vi "Step-3-Top.vi"(9 "Override Iterations":bool=TRUE, 10 "# of Iterations":i32, 11 "input":T1={"a"=[17305248937841088298, 17024460552111218704], "b"=[9581029972675991065, 9654787791092207119], "hp_state_in"=array[2097152 elements], "hp_state_out"=array[2097152 elements], "hp_state_in (u64)"=array[262144 elements], "hp_state_out (u64)"=array[262144 elements]} {"a" format="%.0x"; "b" format="%.0x"; "hp_state_in" format="%.0x"; "hp_state_out" format="%.0x"; "hp_state_in (u64)" format="%.0x"; "hp_state_out (u64)" format="%.0x"}) -> (0 "hp_state out (u64)":u64[](array[numeric]) format="%.0x", 2 "b_out":u64[](array[numeric]) format="%.0x", 3 "a_out":u64[](array[numeric]) format="%.0x")   [LabVIEW 2017]
uses:
  Tests/Helpers/Step-3-Data-Type.ctl
panel:
  out "# of Iterations":i32
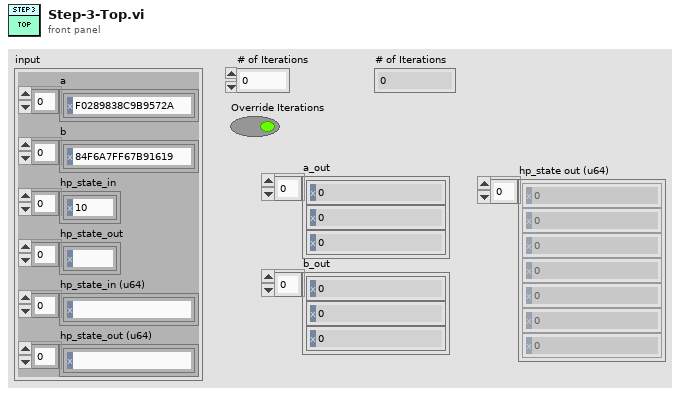
[diagram p1: front panel]
types:
  T1 = typedef "Step-3-Data-Type.ctl" = cluster{"a":u64[], "b":u64[], "hp_state_in":u8[], "hp_state_out":u8[], "hp_state_in (u64)":u64[], "hp_state_out (u64)":u64[]}
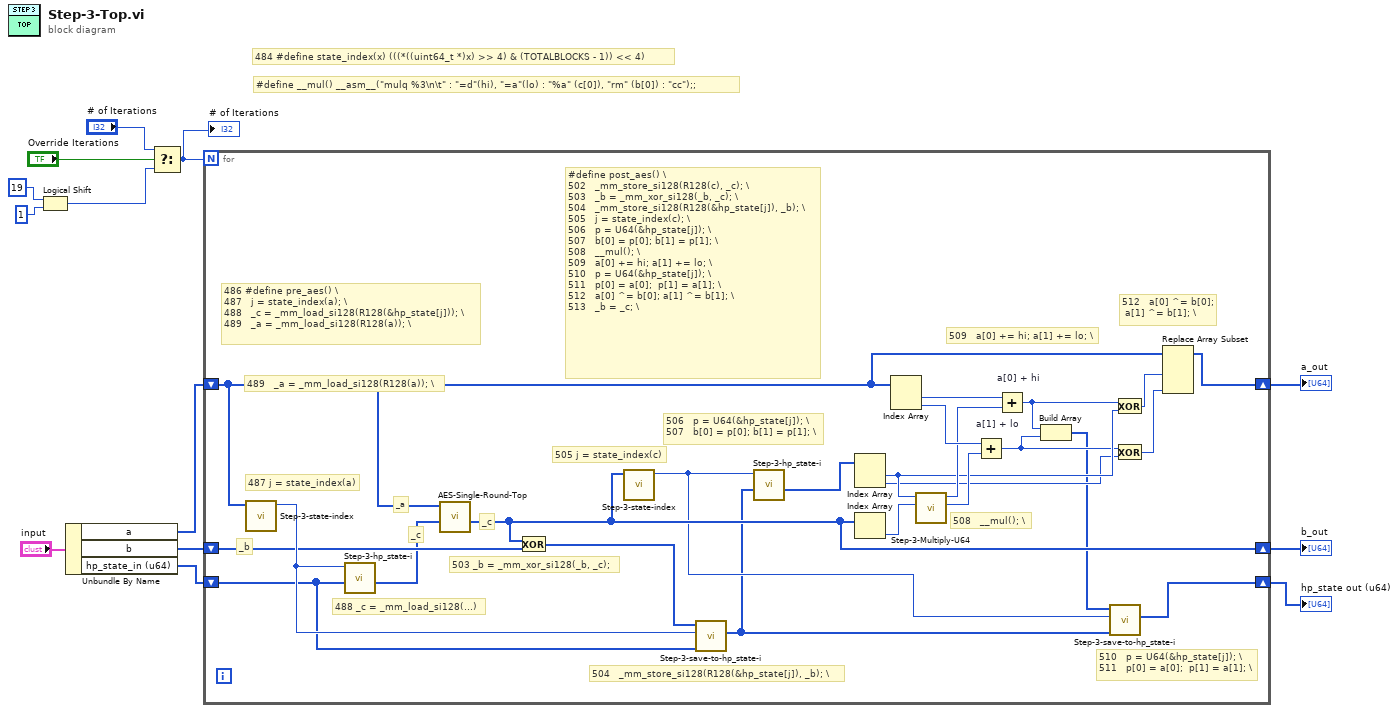
[diagram p0: block diagram]
diagram:
  # "#define __mul() __asm__(\"mulq %3\\n\\t\" : \"=d\"(hi), \"=a\"(lo) : \"%a\" (c[0]), \"rm\" (b[0]) : \"cc\");;"
  # "484 #define state_index(x) (((*((uint64_t *)x) >> 4) & (TOTALBLOCKS - 1)) << 4)"
  n1 = Logical Shift(y=19, x=1) -> (x << y=w6:i32)
  n2 = Unbundle By Name("input") -> ("a"=w11:u64[], "b"=w10:u64[], "hp_state_in (u64)"=w2:u64[])
  n3 = Select(t="# of Iterations", s="Override Iterations", f=w6) -> (s? t:f=w4:i32)
  "# of Iterations" <- w4
  n4 = for {
    N: w4 -> [_]
    shift-right: [w26] -> w9
    shift-left: w10 -> [w29]
    shift-right: [w31] -> w8
    shift-left: w11 -> [w14]
    shift-right: [w17] -> w1
    shift-left: w2 -> [w23]
    # "_c"
    # "_a"
    # "489   _a = _mm_load_si128(R128(a)); \\"
    # "510   p = U64(&hp_state[j]); \\\n511   p[0] = a[0];  p[1] = a[1]; \\"
    # "508   __mul(); \\"
    # "509   a[0] += hi; a[1] += lo; \\"
    # "512   a[0] ^= b[0];\n a[1] ^= b[1]; \\"
    # "506   p = U64(&hp_state[j]); \\\n507   b[0] = p[0]; b[1] = p[1]; \\"
    # "505 j = state_index(c)"
    # "504   _mm_store_si128(R128(&hp_state[j]), _b); \\"
    # "_c"
    # "_b"
    # "503 _b = _mm_xor_si128(_b, _c);"
    # "488 _c = _mm_load_si128(...)"
    # "487 j = state_index(a)"
    # "#define post_aes() \\\n502   _mm_store_si128(R128(c), _c); \\\n503   _b = _mm_xor_si128(_b, _c); \\\n504   _mm_store_si128(R128(&hp_state[j]), _b); \\\n505   j = state_index(c); \\\n506   p = U64(&hp_state[j]); \\\n507   b[0] = p[0]; b[1] = p[1]; \\\n508   __mul(); \\\n509   a[0] += hi; a[1] += lo; \\\n510   p = U64(&hp_state[j]); \\\n511   p[0] = a[0];  p[1] = a[1]; \\\n512   a[0] ^= b[0]; a[1] ^= b[1]; \\\n513   _b = _c; \\"
    # "486 #define pre_aes() \\\n487   j = state_index(a); \\\n488   _c = _mm_load_si128(R128(&hp_state[j])); \\\n489   _a = _mm_load_si128(R128(a)); \\"
    n5 = call "Step-3-state-index.vi"("2 x U64"=w14) -> ("j"=w30:u64)  [unwired: 10 in]
    n6 = call "Step-3-hp_state-i.vi"("hp_state_in (u64)"=w23, "j"=w30) -> ("U64-Array"=w15:u64[])  [unwired: 9 in]
    n7 = call "AES-Single-Round-Top.vi"("state (_c) U64"=w15, "key (_a)"=w14) -> ("state out (c) U64"=w26:u64[])  [unwired: 9 in]
    n8 = Exclusive Or(1:w29, 2:w26) -> (0:w28:u64[])
    n9 = call "Step-3-state-index.vi"("2 x U64"=w26) -> ("j"=w19:u64)  [unwired: 10 in]
    n10 = call "Step-3-save-to-hp_state-i.vi"("hp_state_in (u64)"=w23, "j"=w30, "New-Val"=w28) -> ("hp_state_out (u64)"=w18:u64[])  [unwired: 8 in]
    n11 = call "Step-3-hp_state-i.vi"("hp_state_in (u64)"=w18, "j"=w19) -> ("U64-Array"=w16:u64[])  [unwired: 9 in]
    n12 = Index Array(array=w16) -> (element #1=w25:u64, element #2=w24:u64)  [unwired: 2 in]
    n13 = Index Array(array=w26) -> (element=w27:u64)  [unwired: 1 in]
    n14 = Index Array(array=w14) -> (element #1=w37:u64, element #2=w36:u64)  [unwired: 2 in]
    n15 = call "Step-3-Multiply-U64.vi"("c[0]"=w27, "b[0]"=w25) -> ("lo"=w35:u64, "hi"=w34:u64)  [unwired: 8 in]
    n16 = Add "a[1] + lo"(x=w36, y=w35) -> (x+y=w21:u64)
    n17 = Add "a[0] + hi"(x=w37, y=w34) -> (x+y=w22:u64)
    n18 = Build Array(w22, w21) -> (w20:u64[])
    n19 = call "Step-3-save-to-hp_state-i.vi"("hp_state_in (u64)"=w18, "j"=w19, "New-Val"=w20) -> ("hp_state_out (u64)"=w17:u64[])  [unwired: 8 in]
    n20 = Exclusive Or(1:w25, 2:w22) -> (0:w33:u64)
    n21 = Exclusive Or(1:w24, 2:w21) -> (0:w32:u64)
    n22 = Replace Array Subset(array=w14, new element #1=w33, new element #2=w32) -> (w31:u64[])  [unwired: 2 in]
  }
  "b_out" <- w9
  "a_out" <- w8
  "hp_state out (u64)" <- w1
